vi "HFRR ADV v044.vi"() -> ()   [LabVIEW 2025] (continued)
                n2757 = Multiply(x=w3274, y=w3260) -> (x*y=w3266:dbl)
                n2758 = Subtract(x=w3267, y=w3277) -> (x-y=w3269:dbl)
                n2759 = local read "Save"() -> (w3270:bool)
                n2760 = Add(x=w3269, y=w3266) -> (x+y=w3253:dbl)
                "Elapsed time 3" <- w3253
                n2761 = And(x=w3255, y=w3270) -> (x .and. y?=w3268:bool)
                n2762 = Divide(x=w3253, y=60.0) -> (x/y=w3264:dbl)
                n2763 = local read "Test \nStatus"() -> (w3254:bool)
                n2764 = local read "clk"() -> (w3261:dbl)
                n2765 = Equal?(x=w3261, y=10.0) -> (x = y?=w3263:bool)
                n2766 = case shown="True" w3268 {
                  tunnel: w3267 -> [_ w3394]
                  tunnel: [FALSE ("Boolean 2") TRUE ("Boolean 2")] -> _
                  frame False {
                  }
                  frame True {
                    w3348 = ";" ("Substring")
                    # "Pid out/\nFreq response value"
                    n2767 = local write "act save time"(w3394) -> ()
                    n2768 = local read "FILE"() -> (w3342:string)
                    n2769 = call "file check.vi"("file name in"=w3342) -> ("error out"=w3345:errorcluster, "file name out"=w3340:string)  [unwired: 9 in]
                    n2770 = local read "LVDT STROKE"() -> (w3337:dbl)
                    n2771 = local read "Add up Stroke"() -> (w3335:dbl)
                    n2772 = call "FILE PATH CREATION.vi"("error in"=w3345, "FILE NAME :"=w3340) -> ("FILE OUT"=w3343:path)  [unwired: 8 in, 1 out]
                    n2773 = local read "STROKE Initialize"() -> (w3330:bool)
                    n2774 = Concatenate Strings(w3340, ".dgf" ("Substring")) -> (w3344:string)
                    n2775 = Subtract(x=w3337, y=w3335) -> (x-y=w3336:dbl)
                    n2776 = Absolute Value(x=w3336) -> (abs(x)=w3333:dbl)
                    n2777 = local read "FF 2"() -> (→"Frictional Force ( N )" →"Frictional Force ( N )":dbl)
                    n2778 = Build Path(base path=w3343, name or relative path=w3344) -> (appended path=w3339:path)
                    n2779 = flat-sequence {
                      tunnel: w3333 -> [w3399]
                      tunnel: [w3398] -> w3331
                      tunnel: w3330 -> [w3396]
                      tunnel: [w3401] -> w3332
                      tunnel: w3331 -> [w3401]
                      frame #0 {
                        n2780 = call <vilib>:"Mean PtByPt.vi"("x"=w3399, "sample length"="STROKE FILTER", "initialize"=w3396) -> ("mean"=w3398:dbl)  [unwired: 1 in, 1 out]
                      }
                      frame #1 {
                        "STROKE Initialize" <- FALSE ("STROKE Initialize")
                      }
                    }
                    n2781 = local read "COF 2"() -> (w3353:dbl)
                    "Coefficient of Friction" <- w3353
                    "COF 4" <- w3353
                    "Coefficient of Friction" <- w3353
                    n2782 = local read "TEMP"() -> (w3356:dbl)
                    "Temperature ( Deg C )" <- w3356
                    n2783 = local read "Humidity ( %RH )"() -> (w3355:dbl)
                    n2784 = local read "Frequency ( Hz )"() -> (w3362:dbl)
                    n2785 = local read "LVDT STROKE DISPLAY"() -> (w3334:dbl)
                    n2786 = local read "Elapsed time"() -> (w3387:dbl)
                    n2787 = local read "AIR TEMP"() -> (w3360:dbl)
                    n2788 = local read "PID-out"() -> (w3365:dbl)
                    n2789 = local write "Temperature ( Deg C )"(w3356) -> ()
                    n2790 = Number To Fractional String(number=w3334, width (-)=i16 9 ("precision (6)"), precision (6)=i16 6) -> (F-format string=w3380:string)  [unwired: 1 in]
                    n2791 = Number To Fractional String(number=w3360, width (-)=i16 9 ("precision (6)"), precision (6)=i16 3) -> (F-format string=w3379:string)  [unwired: 1 in]
                    n2792 = Number To Fractional String(number=w3356, width (-)=i16 9 ("precision (6)"), precision (6)=i16 3) -> (F-format string=w3376:string)  [unwired: 1 in]
                    n2793 = Number To Fractional String(number=w3355, width (-)=i16 9 ("precision (6)"), precision (6)=i16 3) -> (F-format string=w3373:string)  [unwired: 1 in]
                    n2794 = Number To Fractional String(number=0.0, width (-)=i16 9 ("precision (6)"), precision (6)=i16 3) -> (F-format string=w3370:string)  [unwired: 1 in]
                    n2795 = Number To Fractional String(number=w3365, width (-)=i16 9 ("precision (6)"), precision (6)=i16 3) -> (F-format string=w3366:string)  [unwired: 1 in]
                    n2796 = Number To Fractional String(number=w3362, width (-)=i16 9 ("precision (6)"), precision (6)=i16 3) -> (F-format string=w3361:string)  [unwired: 1 in]
                    n2797 = Number To Fractional String(number=w3353, width (-)=i16 9 ("precision (6)"), precision (6)=i16 6) -> (F-format string=w3388:string)  [unwired: 1 in]
                    n2798 = Number To Fractional String(number=w3387, width (-)=i16 14 ("precision (6)"), precision (6)=i16 3) -> (F-format string=w3389:string)  [unwired: 1 in]
                    n2799 = Bundle("y"=1.02, "LVDT STROKE DISPLAY"=w3334, "y"=0.98) -> (w3354:T30)  [unwired: 1 in]
                    n2800 = Number To Fractional String(number="Ambient Humidity :", width (-)=i16 9 ("precision (6)"), precision (6)=i16 6) -> (F-format string=w3346:string)  [unwired: 1 in]
                    n2801 = local read "RUN"() -> (w3352:bool)
                    n2802 = case shown="True" w3352 {
                      tunnel: w3354 -> [_ w3405]
                      tunnel: w3334 -> [_ w3404]
                      tunnel: w3334 -> [_ w3402]
                      tunnel: w3334 -> [_ w3403]
                      frame False {
                      }
                      frame True {
                        "Stroke ( mm )" <- w3405
                        "Stroke ( mm )" <- w3405
                        "Stroke 4" <- w3404
                        "Stroke 3" <- w3402
                        "Stroke 2" <- w3403
                        "measured_stroke" <- w3402
                      }
                    }
                    n2803 = Concatenate Strings(w3389, w3348, w3388, w3348, w3380, w3348, w3379, w3348, w3376, w3348, w3373, w3348, w3370, w3348, w3366, w3348, w3361, w3348, w3346, "\r") -> (w3386:string)
                    n2804 = call <vilib>:"Write Characters To File.vi"("append to file? (new file:F)"=TRUE, "character string"=w3386, "file path (dialog if empty)"=w3339) -> ()  [unwired: 2 in, 1 out]
                    "refresh flag" <- TRUE ("refresh flag")
                    "LVDT STROKE Actual" <- w3332
                  }
                }
                n2805 = case shown="True" w3254 {
                  tunnel: w3264 -> [_ w3290]
                  tunnel: w3269 -> [_ w3300]
                  tunnel: [0.0 w3296] -> _
                  tunnel: w3263 -> [_ w3295]
                  tunnel: [0.0 w3294] -> _
                  tunnel: w3253 -> [_ w3294]
                  tunnel: w3267 -> [w3283 _]
                  frame False {
                    n2806 = local write "acq timer"(w3283) -> ()
                    n2807 = local write "Test Duration Status"(0.0 ("Test Duration Status")) -> ()
                  }
                  frame True {
                    n2808 = local read "Set Hz"() -> (w3297:dbl)
                    n2809 = local write "Elapsed time"(w3290) -> ()
                    n2810 = local read "test time"() -> (w3289:dbl)
                    n2811 = Multiply(x=w3300, y=w3297) -> (x*y=w3299:dbl)
                    n2812 = case shown="False" w3295 {
                      tunnel: w3299 -> [w3301 _]
                      tunnel: [w3301 1.0] -> w3296
                      frame False {
                        n2813 = local write "Cycles elapsed"(w3301) -> ()
                      }
                      frame True {
                      }
                    }
                    n2814 = Greater?(x=w3290, y=w3289) -> (0:w3298:bool)
                    n2815 = Subtract(x=w3289, y=w3290) -> (x-y=w3288:dbl)
                    n2816 = Multiply(x=w3288, y=60.0) -> (x*y=w3287:dbl)
                    n2817 = local write "Time Remaining"(w3287) -> ()
                    n2818 = local write "Remaining Time"(w3287) -> ()
                    n2819 = case shown="True" w3298 {
                      frame False {
                      }
                      frame True {
                        n2820 = stacked-sequence {
                          frame #0 {
                            w3306 = T19."Enabled" ("Disabled")
                            w3305 = FALSE ("TEST FILE NAM,E SAVED")
                            w3307 = "" ("FILE")
                            w3308 = TRUE ("Visible")
                            n2821 = local write "Humidity"(FALSE ("Humidity")) -> ()
                            n2822 = local write "RUN"(FALSE ("OK Button 2")) -> ()
                            n2823 = local write "Heater Button"(FALSE ("Heater Button")) -> ()
                            n2824 = local write "Auto Start Test"(FALSE ("Auto Start Test")) -> ()
                            n2825 = local write "TestCompFlg"(TRUE ("StpFlg")) -> ()
                            n2826 = local read "Humidity ( %RH )"() -> (→"Rh After":dbl)
                            n2827 = property on="STOP 2" class="Bool (strict)"("Disabled"=u8 0) -> ()  [unwired: 2 in, 2 out]
                            n2828 = local read "EVENT LOG"() -> (w3313:string)
                            n2829 = call "Event Log.vi"("Content"="Test Completed", "EVENT LOG"=w3313) -> ("EVENT LOG"=w3312:string)  [unwired: 8 in, 1 out]
                            n2830 = property on="RUN" class="Bool (strict)"("Visible"=w3308) -> ()  [unwired: 2 in, 2 out]
                            n2831 = property on="Auto Start Test" class="Bool (strict)"("Visible"=w3308) -> ()  [unwired: 2 in, 2 out]
                            n2832 = local write "Batch Ref Num :"(w3307) -> ()
                            n2833 = local write "FILE"(w3307) -> ()
                            n2834 = local write "EVENT LOG"(w3312) -> ()
                            n2835 = local write "TEST FILE NAM,E SAVED"(w3305) -> ()
                            n2836 = local write "Fuel Discription :"(w3307) -> ()
                            n2837 = local write "START TEMP"(w3305) -> ()
                            n2838 = local write "Remarks :"(w3307) -> ()
                            n2839 = local write "Main Dashboard Buttons"(T1."Imaging" ("Main Dashboard Buttons")) -> ()
                            n2840 = local write "Main Tab"(T4."Adv Scar" ("Main Tab")) -> ()
                            n2841 = property on="FRICVALZ 2" class="Bool (strict)"("DisabledEnum"=w3306) -> ()  [unwired: 2 in, 2 out]
                            n2842 = property on="FRICVALZ 3" class="Bool (strict)"("DisabledEnum"=w3306) -> ()  [unwired: 2 in, 2 out]
                            n2843 = property on="FRICVALZ 4" class="Bool (strict)"("DisabledEnum"=w3306) -> ()  [unwired: 2 in, 2 out]
                          }
                          frame #1 {
                            n2844 = Wait (ms)(milliseconds to wait=u32 2000) -> ()  [unwired: 1 out]
                          }
                          frame #2 {
                            n2845 = local write "Due Write"("VC;0") -> ()
                          }
                          frame #3 {
                            n2846 = Wait (ms)(milliseconds to wait=u32 2000) -> ()  [unwired: 1 out]
                          }
                          frame #4 {
                            n2847 = local write "Due Write"("VC;0") -> ()
                          }
                          frame #5 {
                            n2848 = Wait (ms)(milliseconds to wait=u32 2000) -> ()  [unwired: 1 out]
                          }
                          frame #6 {
                            n2849 = local write "Due Write"("ST;0") -> ()
                          }
                          frame #7 {
                            n2850 = local write "measured_stroke"(0.0 ("measured_stroke")) -> ()
                            n2851 = Wait (ms)(milliseconds to wait=u32 1500) -> ()  [unwired: 1 out]
                          }
                          frame #8 {
                            n2852 = local write "Due Write"("HE;0") -> ()
                            n2853 = local write "Humidity 2"(TRUE ("Humidity")) -> ()
                          }
                        }
                      }
                    }
                    n2854 = Divide(x=w3290, y=w3289) -> (x/y=w3293:dbl)
                    n2855 = Multiply(x=w3293, y=100.0) -> (x*y=w3291:dbl)
                    n2856 = local write "Test Duration Status"(w3291) -> ()
                  }
                }
              }
              frame #2 {
                n2857 = case shown="True" "Heater Button" {
                  tunnel: [0.0 ("output") w3428] -> w3406
                  frame False {
                    w3409 = TRUE ("tmpchk")
                    n2858 = local read "TEMP"() -> (w3410:dbl)
                    n2859 = local write "Temp ini"(w3410) -> ()
                    n2860 = local write "Reset 4"(w3409) -> ()
                    n2861 = local write "tmpchk"(w3409) -> ()
                    n2862 = local write "reinit"(TRUE ("reinit")) -> ()
                    n2863 = local write "manual temp log"(TRUE ("manual temp log")) -> ()
                  }
                  frame True {
                    # "Logic to turn off\nthe heater when \ntemp is not rising.\nTime - 60 sec\nDelta t- 5°c"
                    n2864 = local read "Temp ini"() -> (w3417:dbl)
                    n2865 = local read "Auto Start Test"() -> (w3413:bool)
                    n2866 = Less?(x=w3417, y=53.0) -> (x < y?=w3415:bool)
                    n2867 = case shown="False" w3413 {
                      frame False {
                        n2868 = local read "Set Temp"() -> (w3437:dbl)
                        n2869 = local read "TEMP"() -> (w3436:dbl)
                        n2870 = Subtract(x=w3437, y=w3436) -> (x-y=w3435:dbl)
                        n2871 = Absolute Value(x=w3435) -> (abs(x)=w3434:dbl)
                        n2872 = Less?(x=w3434, y=0.5) -> (x < y?=w3432:bool)
                        n2873 = case shown="True" w3432 {
                          tunnel: "manual temp log" -> [_ w3438]
                          frame False {
                          }
                          frame True {
                            n2874 = case shown="True" w3438 {
                              selector: w3438 -> [_ w3439]
                              frame False {
                              }
                              frame True {
                                # "#Event log"
                                n2875 = Not(x=w3439) -> (.not. x?=w3440:bool)
                                n2876 = local write "manual temp log"(w3440) -> ()
                                n2877 = local read "EVENT LOG"() -> (w3443:string)
                                n2878 = call "Event Log.vi"("Content"="Target Temperature reached", "EVENT LOG"=w3443) -> ("EVENT LOG"=w3442:string)  [unwired: 8 in, 1 out]
                                n2879 = local write "EVENT LOG"(w3442) -> ()
                              }
                            }
                          }
                        }
                      }
                      frame True {
                        n2880 = local write "manual temp log"(TRUE ("manual temp log")) -> ()
                      }
                    }
                    n2881 = And(x="tmpchk", y=w3415) -> (x .and. y?=w3418:bool)
                    n2882 = case shown="True" w3418 {
                      frame False {
                      }
                      frame True {
                        n2883 = call "Elapsed Time8"("Time Target (s)"=300.0, "Reset"="Reset 4") -> ("Time has Elapsed"=w3445:bool)  [unwired: 10 in, 7 out]
                        n2884 = flat-sequence {
                          tunnel: w3445 -> [_]
                          frame #0 {
                            n2885 = local write "Reset 4"(FALSE ("Reset 4")) -> ()
                          }
                        }
                        n2886 = case shown="True" w3445 {
                          frame False {
                          }
                          frame True {
                            n2887 = local read "Temp ini"() -> (w3452:dbl)
                            n2888 = Add(x=w3452, y=5.0) -> (x+y=w3450:dbl)
                            n2889 = local read "TEMP"() -> (w3453:dbl)
                            n2890 = Greater?(x=w3453, y=w3450) -> (0:w3451:bool)
                            n2891 = case shown="False" w3451 {
                              frame False {
                                n2892 = local write "Heater Button"(FALSE ("Heater Button")) -> ()
                              }
                              frame True {
                                n2893 = local write "tmpchk"(FALSE ("tmpchk")) -> ()
                              }
                            }
                          }
                        }
                      }
                    }
                    n2894 = local read "Set Temp"() -> (w3426:dbl)
                    n2895 = local read "TEMP"() -> (w3420:dbl)
                    n2896 = call-poly <vilib>:"PID.vi"("reinitialize? (F)"="reinit", "dt (s)"=-1.0, "process variable"=w3420, "setpoint"=w3426) -> ("output"=w3423:dbl)  [unwired: 6 in, 1 out]
                    n2897 = Subtract(x=w3426, y=w3420) -> (x-y=w3427:dbl)
                    n2898 = Add(x=w3426, y=0.5) -> (x+y=w3424:dbl)
                    n2899 = Greater Or Equal?(x=w3420, y=w3424) -> ()  [unwired: 1 out]
                    n2900 = Select(t=0.0, s=FALSE, f=w3423) -> (s? t:f=w3422:dbl)
                    "PID output" <- w3422
                    n2901 = flat-sequence {
                      tunnel: w3422 -> [w3456]
                      tunnel: [w3456] -> w3428
                      frame #0 {
                        n2902 = local write "reinit"(FALSE ("reinit")) -> ()
                      }
                    }
                    n2903 = Bundle(w3427, "output"=w3422, "TEMP"=w3420) -> ()  [unwired: 1 in, 1 out]
                  }
                }
                "PID-out" <- w3406
              }
              frame #3 {
                n2904 = local read "TEMP"() -> (w3458:dbl)
                n2905 = Greater Or Equal?(x=w3458, y="Set Temp 2") -> (x >= y?=w3463:bool)
                n2906 = case shown="True" w3463 {
                  tunnel: [FALSE TRUE] -> w3461
                  frame False {
                  }
                  frame True {
                  }
                }
                "Status 13" <- w3461
                n2907 = And(x=w3461, y="trip1 8") -> (x .and. y?=w3460:bool)
                n2908 = case shown="True" w3460 {
                  frame False {
                    n2909 = local write "Heater Trip Temp"(TRUE ("Heater Trip Temp")) -> ()
                  }
                  frame True {
                    w3466 = FALSE ("OK Button 2")
                    n2910 = case shown="True" "Heater Trip Temp" {
                      selector: "Heater Trip Temp" -> [_ w3468]
                      frame False {
                      }
                      frame True {
                        n2911 = Not(x=w3468) -> (.not. x?=w3467:bool)
                        n2912 = local read "EVENT LOG"() -> (w3471:string)
                        n2913 = local write "Heater Trip Temp"(w3467) -> ()
                        n2914 = call "Event Log.vi"("Content"="Heater Trip", "EVENT LOG"=w3471) -> ("EVENT LOG"=w3470:string)  [unwired: 8 in, 1 out]
                        n2915 = local write "EVENT LOG"(w3470) -> ()
                      }
                    }
                    n2916 = local write "RUN"(w3466) -> ()
                    n2917 = property on="Auto Start Test" class="Bool (strict)"("Value"=w3466) -> ()  [unwired: 2 in, 2 out]
                    n2918 = local write "Heater Button"(w3466) -> ()
                  }
                }
              }
            }
            n2919 = case shown="False" w3177 {
              frame False {
                n2920 = disable-structure shown="Disabled" {
                  frame Disabled {
                    n2921 = stacked-sequence {
                      frame #0 {
                        n2922 = local write "RUN"(FALSE ("OK Button 2")) -> ()
                      }
                      frame #1 {
                      }
                    }
                  }
                  frame Enabled {
                  }
                }
              }
              frame True {
              }
            }
          }
        }
        n2923 = local read "Reset Graph"() -> (w3074:bool)
        n2924 = case shown="True" w3074 {
          selector: w3074 -> [_ w3091]
          frame False {
          }
          frame True {
            w3105 = 0.0 ("X Scale.Range:Maximum")
            n2925 = Not(x=w3091) -> (.not. x?=w3090:bool)
            n2926 = local write "Reset Graph"(w3090) -> ()
            n2927 = property on="Electrical Contact Resistance ( % )" class="WFChart (strict)"("XScale.Maximum"=600.0 ("X Scale.Range:Maximum"), "XScale.Minimum"=0.0 ("X Scale.Range:Minimum"), "YScale.Maximum"=100.0 ("Y Scale.Range:Maximum"), "YScale.Minimum"=0.0 ("Y Scale.Range:Minimum")) -> ()  [unwired: 2 in, 2 out]
            n2928 = property on="Frictional Force ( N )" class="WFChart (strict)"("XScale.Maximum"=600.0 ("X Scale.Range:Maximum"), "XScale.Minimum"=0.0 ("X Scale.Range:Minimum"), "YScale.Maximum"=100.0 ("Y Scale.Range:Maximum"), "YScale.Minimum"=0.0 ("Y Scale.Range:Minimum")) -> ()  [unwired: 2 in, 2 out]
            n2929 = property on="Temperature ( Deg C )" class="WFChart (strict)"("XScale.Maximum"=600.0 ("X Scale.Range:Maximum"), "XScale.Minimum"=0.0 ("X Scale.Range:Minimum"), "YScale.Maximum"=100.0 ("Y Scale.Range:Maximum"), "YScale.Minimum"=0.0 ("Y Scale.Range:Minimum")) -> ()  [unwired: 2 in, 2 out]
            n2930 = property on="Stroke ( mm )" class="WFChart (strict)"("XScale.Maximum"=600.0 ("X Scale.Range:Maximum"), "XScale.Minimum"=0.0 ("X Scale.Range:Minimum"), "YScale.Maximum"=100.0 ("Y Scale.Range:Maximum"), "YScale.Minimum"=0.0 ("Y Scale.Range:Minimum")) -> ()  [unwired: 2 in, 2 out]
            n2931 = property on="Coefficient of Friction" class="WFChart (strict)"("XScale.Maximum"=600.0 ("X Scale.Range:Maximum"), "XScale.Minimum"=0.0 ("X Scale.Range:Minimum"), "YScale.Maximum"=100.0 ("Y Scale.Range:Maximum"), "YScale.Minimum"=0.0 ("Y Scale.Range:Minimum")) -> ()  [unwired: 2 in, 2 out]
            n2932 = property on="Electrical Contact Resistance ( % )" class="WFChart (strict)"("XScale.Minimum"=0.0 ("X Scale.Range:Minimum"), "XScale.Maximum"=600.0 ("X Scale.Range:Maximum"), "YScale.Minimum"=0.0 ("Y Scale.Range:Minimum"), "YScale.Maximum"=100.0 ("Y Scale.Range:Maximum")) -> ()  [unwired: 2 in, 2 out]
            n2933 = property on="Temperature ( Deg C )" class="WFChart (strict)"("XScale.Minimum"=0.0 ("X Scale.Range:Minimum"), "XScale.Maximum"=600.0 ("X Scale.Range:Maximum"), "YScale.Minimum"=0.0 ("Y Scale.Range:Minimum"), "YScale.Maximum"=100.0 ("Y Scale.Range:Maximum")) -> ()  [unwired: 2 in, 2 out]
            n2934 = property on="Coefficient of Friction" class="WFChart (strict)"("XScale.Minimum"=0.0 ("X Scale.Range:Minimum"), "XScale.Maximum"=600.0 ("X Scale.Range:Maximum"), "YScale.Maximum"=1.0 ("X Scale.Range:Minimum"), "YScale.Minimum"=0.0 ("X Scale.Range:Minimum")) -> ()  [unwired: 2 in, 2 out]
            n2935 = property on="Frictional Force ( N )" class="WFChart (strict)"("XScale.Maximum"=600.0 ("X Scale.Range:Maximum"), "XScale.Minimum"=w3105, "YScale.Maximum"=10.0 ("Y Scale.Range:Maximum"), "YScale.Minimum"=w3105) -> ()  [unwired: 2 in, 2 out]
            n2936 = property on="Stroke ( mm )" class="WFChart (strict)"("XScale.Maximum"=600.0 ("X Scale.Range:Maximum"), "XScale.Minimum"=0.0 ("X Scale.Range:Minimum"), "YScale.Maximum"=100.0 ("Y Scale.Range:Maximum"), "YScale.Minimum"=0.0 ("Y Scale.Range:Minimum")) -> ()  [unwired: 2 in, 2 out]
          }
        }
      }
      frame "Compare Files" {
        # "Elapsed time\ncof\nstroke\nAir temp\nTemp\nHumidity"
        n2937 = case shown="True" "RSTV1 2" {
          frame False {
          }
          frame True {
            n2938 = property on="Humidity ( %RH )" class="XYGraph (strict)"("Y Scale.Display Format:Precision"=u8 0 ("Y Scale.Format & Precision:Precision")) -> ()  [unwired: 2 in, 2 out]
            n2939 = property on="Humidity ( %RH )" class="XYGraph (strict)"("X Scale.Range:Minimum"=0.0, "X Scale.Range:Maximum"=75.0, "Y Scale.Range:Minimum"=48.0, "Y Scale.Range:Maximum"=58.0) -> ()  [unwired: 2 in, 2 out]
          }
        }
        n2940 = case shown="True" "RST CP 2" {
          frame False {
          }
          frame True {
            n2941 = property on="XY Graph 13" class="XYGraph (strict)"("Y Scale.Display Format:Precision"=u8 0 ("Y Scale.Format & Precision:Precision")) -> ()  [unwired: 2 in, 2 out]
            n2942 = property on="XY Graph 13" class="XYGraph (strict)"("X Scale.Range:Minimum"=0.0, "X Scale.Range:Maximum"=75.0, "Y Scale.Range:Minimum"=0.0, "Y Scale.Range:Maximum"=100.0) -> ()  [unwired: 2 in, 2 out]
          }
        }
        n2943 = case shown="True" "RST CP" {
          frame False {
          }
          frame True {
            n2944 = property on="Sample Temperature ( °C )" class="XYGraph (strict)"("Y Scale.Display Format:Precision"=u8 2 ("Y Scale.Format & Precision:Precision")) -> ()  [unwired: 2 in, 2 out]
            n2945 = property on="Sample Temperature ( °C )" class="XYGraph (strict)"("X Scale.Range:Minimum"=0.0, "X Scale.Range:Maximum"=75.0, "Y Scale.Range:Minimum"=58.0, "Y Scale.Range:Maximum"=62.0) -> ()  [unwired: 2 in, 2 out]
          }
        }
        n2946 = case shown="True" "RSTV1 3" {
          frame False {
          }
          frame True {
            n2947 = property on="Air Temperature  ( °C )" class="XYGraph (strict)"("Y Scale.Display Format:Precision"=u8 2 ("Y Scale.Format & Precision:Precision")) -> ()  [unwired: 2 in, 2 out]
            n2948 = property on="Air Temperature  ( °C )" class="XYGraph (strict)"("X Scale.Range:Minimum"=0.0 ("Y Scale.Range:Minimum"), "X Scale.Range:Maximum"=75.0 ("Y Scale.Range:Maximum"), "Y Scale.Range:Minimum"=20.0 ("X Scale.Range:Minimum"), "Y Scale.Range:Maximum"=26.0 ("X Scale.Range:Maximum")) -> ()  [unwired: 2 in, 2 out]
          }
        }
        n2949 = case shown="True" "RSTV1 4" {
          frame False {
          }
          frame True {
            n2950 = property on="Stroke ( mm )" class="XYGraph (strict)"("Y Scale.Display Format:Precision"=u8 2 ("Y Scale.Format & Precision:Precision")) -> ()  [unwired: 2 in, 2 out]
            n2951 = property on="Stroke ( mm )" class="XYGraph (strict)"("X Scale.Range:Minimum"=0.0 ("Y Scale.Range:Maximum"), "X Scale.Range:Maximum"=75.0 ("X Scale.Range:Minimum"), "Y Scale.Range:Minimum"=0.98, "Y Scale.Range:Maximum"=1.02) -> ()  [unwired: 2 in, 2 out]
          }
        }
        n2952 = case shown="True" "rstv2" {
          frame False {
          }
          frame True {
            n2953 = property on="Coefficient Of Friction" class="XYGraph (strict)"("Y Scale.Display Format:Precision"=u8 3 ("Y Scale.Format & Precision:Precision")) -> ()  [unwired: 2 in, 2 out]
            n2954 = property on="Coefficient Of Friction" class="XYGraph (strict)"("X Scale.Range:Minimum"=0.0 ("Y Scale.Range:Maximum"), "X Scale.Range:Maximum"=75.0, "Y Scale.Range:Minimum"=0.0, "Y Scale.Range:Maximum"=1.0 ("X Scale.Range:Minimum")) -> ()  [unwired: 2 in, 2 out]
          }
        }
        n2955 = case shown="True" "RST CP 3" {
          frame False {
          }
          frame True {
            n2956 = property on="Air Temp ( °C ) vs Humidity ( % RH )" class="XYGraph (strict)"("X Scale.Range:Minimum"=18.0, "X Scale.Range:Maximum"=28.0 ("X Scale.Range:Minimum"), "Y Scale.Range:Minimum"=30.0 ("X Scale.Range:Minimum"), "Y Scale.Range:Maximum"=70.0 ("X Scale.Range:Minimum")) -> ()  [unwired: 2 in, 2 out]
          }
        }
        n2957 = case shown="True" "OPEN 1" {
          frame False {
          }
          frame True {
            (unwired) 0  # existing file
            w3747 = "Choose a datalog file to open"  # prompt
            n2958 = local write "OPEN 1"(FALSE ("OPEN 1")) -> ()
            n2959 = String To Path(string="C:\\LAB-IQ\\Data\\") -> (path=w3732:path)
            n2960 = File Dialog(6:"*.dgf" ("pattern"), 7:w3747, 11:w3732) -> (0:w3730:errorcluster, 3:w3738:path)  [unwired: 4 in, 2 out]
            n2961 = Unbundle(w3730) -> ()  [unwired: 3 out]
            n2962 = Strip Path(path=w3738) -> (name=w3737:string)  [unwired: 1 out]
            n2963 = Path To String(path=w3738) -> (string=w3733:string)
            "string1" <- w3733
            n2964 = Match Pattern(string=w3737, regular expression=".dgf") -> (before substring=→"String Control":string)  [unwired: 1 in, 3 out]
            n2965 = Match Pattern(string=w3733, regular expression=".dgf" ("substring (\"\")")) -> (before substring=w3743:string)  [unwired: 1 in, 3 out]
            n2966 = Concatenate Strings(w3743, ".duf" ("Substring")) -> (w3739:string)
            n2967 = String To Path(string=w3739) -> (path=w3744:path)
            n2968 = call <vilib>:"Read Characters From File.vi"("file path (dialog if empty)"=w3744, "start of read offset (chars.:0)"=60 ("start of read offset (chars.: 0)")) -> ("character string"=→"String Control 2":string)  [unwired: 4 in, 3 out]
          }
        }
        n2969 = case shown="True" "OPEN 2" {
          frame False {
          }
          frame True {
            (unwired) 0  # existing file
            w3765 = "Choose a datalog file to open"  # prompt
            n2970 = local write "OPEN 2"(FALSE ("OPEN 1")) -> ()
            n2971 = String To Path(string="C:\\LAB-IQ\\Data\\") -> (path=w3750:path)
            n2972 = File Dialog(6:"*.dgf" ("pattern"), 7:w3765, 11:w3750) -> (0:w3748:errorcluster, 3:w3756:path)  [unwired: 4 in, 2 out]
            n2973 = Unbundle(w3748) -> ()  [unwired: 3 out]
            n2974 = Strip Path(path=w3756) -> (name=w3754:string)  [unwired: 1 out]
            n2975 = Path To String(path=w3756) -> (string=w3751:string)
            "string1 2" <- w3751
            n2976 = Match Pattern(string=w3754, regular expression=".dgf") -> (before substring=→"String Control 3":string)  [unwired: 1 in, 3 out]
            n2977 = Match Pattern(string=w3751, regular expression=".dgf" ("substring (\"\")")) -> (before substring=w3762:string)  [unwired: 1 in, 3 out]
            n2978 = Concatenate Strings(w3762, ".duf" ("Substring")) -> (w3759:string)
            n2979 = String To Path(string=w3759) -> (path=w3757:path)
            n2980 = call <vilib>:"Read Characters From File.vi"("file path (dialog if empty)"=w3757, "start of read offset (chars.:0)"=60 ("start of read offset (chars.: 0)")) -> ("character string"=→"String Control 4":string)  [unwired: 4 in, 3 out]
          }
        }
        n2981 = case shown="True" "OPEN 3" {
          frame False {
          }
          frame True {
            (unwired) 0  # existing file
            w3783 = "Choose a datalog file to open"  # prompt
            n2982 = local write "OPEN 3"(FALSE ("OPEN 1")) -> ()
            n2983 = String To Path(string="C:\\LAB-IQ\\Data\\") -> (path=w3768:path)
            n2984 = File Dialog(6:"*.dgf" ("pattern"), 7:w3783, 11:w3768) -> (0:w3766:errorcluster, 3:w3774:path)  [unwired: 4 in, 2 out]
            n2985 = Unbundle(w3766) -> ()  [unwired: 3 out]
            n2986 = Strip Path(path=w3774) -> (name=w3772:string)  [unwired: 1 out]
            n2987 = Path To String(path=w3774) -> (string=w3769:string)
            "string1 3" <- w3769
            n2988 = Match Pattern(string=w3772, regular expression=".dgf") -> (before substring=→"String Control 5":string)  [unwired: 1 in, 3 out]
            n2989 = Match Pattern(string=w3769, regular expression=".dgf" ("substring (\"\")")) -> (before substring=w3779:string)  [unwired: 1 in, 3 out]
            n2990 = Concatenate Strings(w3779, ".duf" ("Substring")) -> (w3776:string)
            n2991 = String To Path(string=w3776) -> (path=w3780:path)
            n2992 = call <vilib>:"Read Characters From File.vi"("file path (dialog if empty)"=w3780, "start of read offset (chars.:0)"=60 ("start of read offset (chars.: 0)")) -> ("character string"=→"String Control 6":string)  [unwired: 4 in, 3 out]
          }
        }
        n2993 = case shown="True" "OPEN 4" {
          frame False {
          }
          frame True {
            (unwired) 0  # existing file
            w3801 = "Choose a datalog file to open"  # prompt
            n2994 = local write "OPEN 4"(FALSE ("OPEN 1")) -> ()
            n2995 = String To Path(string="C:\\LAB-IQ\\Data\\") -> (path=w3786:path)
            n2996 = File Dialog(6:"*.dgf" ("pattern"), 7:w3801, 11:w3786) -> (0:w3784:errorcluster, 3:w3792:path)  [unwired: 4 in, 2 out]
            n2997 = Unbundle(w3784) -> ()  [unwired: 3 out]
            n2998 = Strip Path(path=w3792) -> (name=w3790:string)  [unwired: 1 out]
            n2999 = Path To String(path=w3792) -> (string=w3787:string)
            "string1 4" <- w3787
            n3000 = Match Pattern(string=w3790, regular expression=".dgf") -> (before substring=→"String Control 7":string)  [unwired: 1 in, 3 out]
            n3001 = Match Pattern(string=w3787, regular expression=".dgf" ("substring (\"\")")) -> (before substring=w3797:string)  [unwired: 1 in, 3 out]
            n3002 = Concatenate Strings(w3797, ".duf" ("Substring")) -> (w3794:string)
            n3003 = String To Path(string=w3794) -> (path=w3798:path)
            n3004 = call <vilib>:"Read Characters From File.vi"("file path (dialog if empty)"=w3798, "start of read offset (chars.:0)"=60 ("start of read offset (chars.: 0)")) -> ("character string"=→"String Control 8":string)  [unwired: 4 in, 3 out]
          }
        }
      }
      frame "About" {
        # "Elapsed time\ncof\nstroke\nmean pos\nTemp\nHumidity"
        n3005 = disable-structure shown="Disabled" {
          frame Disabled {
            n3006 = case shown="True" "Export" {
              frame False {
              }
              frame True {
                w3823 = "                                      " ("string")
                w3825 = "\r"
                (unwired) i16 6 ("width (-)")
                w3902 = "\r"
                w3834 = "\r"
                n3007 = local write "Export"(FALSE ("Export")) -> ()
                n3008 = local read "String 29"() -> (w3871:string)
                n3009 = local read "String 34"() -> (w3859:string)
                n3010 = local read "String 35"() -> (w3854:string)
                n3011 = local read "String 37"() -> (w3850:string)
                n3012 = local read "String 36"() -> (w3847:string)
                n3013 = local read "String 38"() -> (w3844:string)
                n3014 = local read "String 39"() -> (w3841:string)
                n3015 = Match Pattern(string=w3871, regular expression=".dwm") -> (before substring=w3867:string)  [unwired: 1 in, 3 out]
                "before substring" <- w3867
                n3016 = local read "S 38"() -> (w3862:string)
                n3017 = local read "S 39"() -> (w3855:string)
                n3018 = local read "Temperature before test 2"() -> (w3891:dbl)
                n3019 = local read "Temperature after test 2"() -> (w3896:dbl)
                n3020 = local read "Humidity before test 2"() -> (w3877:dbl)
                n3021 = local read "Humidity after test 2"() -> (w3892:dbl)
                n3022 = local read "MWSD 2"() -> (w3888:dbl)
                n3023 = local read "WS1.4 2"() -> (w3904:dbl)
                n3024 = local read "HCF 2"() -> (w3900:dbl)
                n3025 = local read "AVP 2"() -> (w3889:dbl)
                n3026 = Concatenate Strings("1," ("string"), w3862) -> (w3861:string)
                n3027 = Concatenate Strings("2," ("string"), w3859) -> (w3858:string)
                n3028 = Concatenate Strings("3," ("string"), w3855) -> (w3857:string)
                n3029 = Concatenate Strings("4," ("string"), w3854) -> (w3853:string)
                n3030 = Concatenate Strings("5," ("string"), w3850) -> (w3851:string)
                n3031 = Concatenate Strings("6," ("string"), w3847) -> (w3848:string)
                n3032 = Concatenate Strings("7," ("string"), w3844) -> (w3845:string)
                n3033 = Concatenate Strings("8," ("string"), w3841) -> (w3842:string)
                n3034 = local read "Sample ID"() -> (w3909:string)
                n3035 = case shown="\"xlx\"" "Select File Type" {
                  tunnel: w3867 -> [w3912 w3914 w3916]
                  tunnel: [w3910 w3915 w3917] -> w3866
                  frame "xlx" {
                    n3036 = Concatenate Strings(w3912, ".xls" ("string")) -> (w3910:string)
                  }
                  frame "csv" {
                    n3037 = Concatenate Strings(w3914, ".csv" ("string")) -> (w3915:string)
                  }
                  frame "txt" {
                    n3038 = Concatenate Strings(w3916, ".txt" ("string")) -> (w3917:string)
                  }
                }
                n3039 = local read "Test Date"() -> (w3908:string)
                n3040 = local read "String 45"() -> (w3822:string)
                n3041 = local read "String 31"() -> (w3907:string)
                n3042 = local read "String 32"() -> (w3906:string)
                n3043 = local read "TITTLE"() -> (w3830:string)
                n3044 = Number To Fractional String(number=w3877, width (-)=i16 6, precision (6)=i16 2) -> (F-format string=w3876:string)  [unwired: 1 in]
                n3045 = Number To Fractional String(number=w3891, width (-)=i16 6, precision (6)=i16 2) -> (F-format string=w3897:string)  [unwired: 1 in]
                n3046 = Number To Fractional String(number=w3892, width (-)=i16 6, precision (6)=i16 2) -> (F-format string=w3890:string)  [unwired: 1 in]
                n3047 = Number To Fractional String(number=w3896, width (-)=i16 6, precision (6)=i16 2) -> (F-format string=w3895:string)  [unwired: 1 in]
                n3048 = Number To Fractional String(number=w3888, width (-)=i16 6, precision (6)=i16 2) -> (F-format string=w3886:string)  [unwired: 1 in]
                n3049 = Number To Fractional String(number=w3889, width (-)=i16 6, precision (6)=i16 2) -> (F-format string=w3887:string)  [unwired: 1 in]
                n3050 = Number To Fractional String(number=w3900, width (-)=i16 6, precision (6)=i16 2) -> (F-format string=w3901:string)  [unwired: 1 in]
                n3051 = Number To Fractional String(number=w3904, precision (6)=i16 2) -> (F-format string=w3905:string)  [unwired: 2 in]
                n3052 = local read "s.NO"() -> (w3824:string)
                n3053 = Concatenate Strings("=" ("string"), w3830) -> (w3829:string)
                n3054 = Concatenate Strings("S.No," ("string"), "                                       Parameters" ("string")) -> (w3835:string)
                n3055 = Concatenate Strings(w3902, w3861, w3876, w3902, w3858, w3897, w3902, w3857, w3890, w3902, w3853, w3895, w3902, w3851, w3886, w3902, w3848, w3887, w3902, w3845, w3901, w3902, w3842, w3905) -> (w3864:string)
                n3056 = Concatenate Strings(w3834, "," ("string"), w3822, w3824, w3823, w3906, w3909, w3823, w3907, w3908, w3834) -> (w3832:string)
                n3057 = local read "Tested by"() -> (w3838:string)
                n3058 = local read "String 33"() -> (w3839:string)
                n3059 = Concatenate Strings("," ("string"), "                                                                             " ("string")) -> (w3827:string)
                n3060 = Concatenate Strings(w3829, w3825, w3832, w3825, w3835, w3864, w3825, w3827, w3839, w3838) -> (→"export":string)
                n3061 = String To Path(string=w3866) -> (path=w3873:path)
                n3062 = local read "export"() -> (w3868:string)
                n3063 = call <vilib>:"Write Characters To File.vi"("append to file? (new file:F)"=FALSE, "character string"=w3868, "file path (dialog if empty)"=w3873) -> ()  [unwired: 2 in, 1 out]
              }
            }
          }
          frame Enabled {
          }
        }
        n3064 = case shown="True" "OK Button 17" {
          frame False {
          }
          frame True {
            (unwired) 0  # existing file
            w4126 = "Choose a datalog file to open"  # prompt
            n3065 = local write "OK Button 17"(FALSE ("OK Button 17")) -> ()
            n3066 = local read "String"() -> (w4121:string)
            n3067 = String To Path(string=w4121) -> (path=w4122:path)
            n3068 = File Dialog(6:"*.duf" ("pattern"), 7:w4126, 11:w4122) -> (0:w4113:errorcluster, 3:w4132:path)  [unwired: 4 in, 2 out]
            n3069 = Unbundle(w4113) -> ()  [unwired: 3 out]
            n3070 = Open/Create/Replace File "Open File"(file path (use dialog)=w4132) -> (refnum out=w4124:refnum<file>)  [unwired: 5 in, 2 out]
            n3071 = Strip Path(path=w4132) -> (name=w4130:string)  [unwired: 1 out]
            n3072 = Path To String(path=w4132) -> (string=w4115:string)
            n3073 = while {
              tunnel: w4124 -> [w4136]
              i -> [w4133]
              stop <- w4134 continue-if-true
              (unwired) TRUE ("line mode (F)")
              n3074 = Read from Text File "Read File"(file (use dialog)=w4136) -> (text=w4135:string)  [unwired: 3 in, 3 out]
              n3075 = local write "Numeric 16"(w4133) -> ()
              n3076 = String Length(string=w4135) -> (length=w4138:i32)
              n3077 = Greater?(x=w4138, y=1) -> (0:w4134:bool)
            }
            n3078 = local write "String 29"(w4115) -> ()
            n3079 = Search and Replace String(input string=w4115, search string=".duf", replace string=".dgf" ("replace string (\"\")")) -> (result string=→"String Indicator 4":string)  [unwired: 5 in, 3 out]
            n3080 = Match Pattern(string=w4130, regular expression=".dwm") -> (before substring=w4114:string)  [unwired: 1 in, 3 out]
            "String Indicator" <- w4114
            n3081 = Match Pattern(string=w4115, regular expression=".dwm" ("substring (\"\")")) -> (before substring=w4116:string)  [unwired: 1 in, 3 out]
            "String Indicator 3" <- w4116
            n3082 = local write "TITTLE 2"(w4114) -> ()
            n3083 = String To Path(string=w4116) -> (path=w4123:path)
            "path" <- w4123
            n3084 = call <vilib>:"Read Characters From File.vi"("file path (dialog if empty)"=w4123, "start of read offset (chars.:0)"=60 ("start of read offset (chars.: 0)")) -> ("character string"=→"String Indicator 2":string)  [unwired: 4 in, 3 out]
          }
        }
        n3085 = call <vilib>:"Query Available Printers.vi"() -> ("system configured printers"=w3815:string[])  [unwired: 9 in, 2 out]
        "System Configured Printers 2" <- w3815
        n3086 = local read "OK Button 16"() -> (w3812:bool)
        n3087 = case shown="True" "OK Button 16" {
          frame False {
          }
          frame True {
            n3088 = stacked-sequence {
              frame #0 {
                n3089 = local read "Numeric 16"() -> (w4140:i32)
                n3090 = local write "Numeric 10"(w4140) -> ()
              }
              frame #1 {
                n3091 = local read "String 29"() -> (w4143:string)
                n3092 = String To Path(string=w4143) -> (path=w4142:path)
                n3093 = Open/Create/Replace File "Open File"(file path (use dialog)=w4142) -> (refnum out=w4144:refnum<file>)  [unwired: 5 in, 2 out]
                n3094 = for {
                  N: 16 -> [_]
                  tunnel: w4144 -> [w4151]
                  i -> [w4147]
                  (unwired) TRUE ("line mode (F)")
                  n3095 = Read from Text File "Read File"(file (use dialog)=w4151) -> (text=w4145:string)  [unwired: 3 in, 3 out]
                  n3096 = Match Pattern(string=w4145, regular expression="(") -> (after substring=w4150:string)  [unwired: 1 in, 3 out]
                  n3097 = Match Pattern(string=w4150, regular expression=")") -> (before substring=w4146:string)  [unwired: 1 in, 3 out]
                  n3098 = case shown="1" w4147 {
                    tunnel: w4146 -> [w4152 w4153 _ _ w4154 w4155 w4156 w4158 w4160 w4162 w4164 w4166 w4168 w4170 _]
                    tunnel: w4145 -> [_ _ _ _ _ _ _ _ _ _ _ _ _ _ _]
                    frame 0 {
                      "TITTLE" <- w4152
                    }
                    frame 1 {
                      "Sample ID" <- w4153
                    }
                    frame 2 {
                    }
                    frame 3 {
                    }
                    frame 4 {
                      "Test Date" <- w4154
                    }
                    frame 5 {
                      "Tested by" <- w4155
                    }
                    frame 6 {
                      n3099 = Fract/Exp String To Number(string=w4156) -> (number=→"Humidity before test 2":dbl)  [unwired: 3 in, 1 out]
                    }
                    frame 7 {
                      n3100 = Fract/Exp String To Number(string=w4158) -> (number=→"Temperature before test 2":dbl)  [unwired: 3 in, 1 out]
                    }
                    frame 8 {
                      n3101 = Fract/Exp String To Number(string=w4160) -> (number=→"Humidity after test 2":dbl)  [unwired: 3 in, 1 out]
                    }
                    frame 9 {
                      n3102 = Fract/Exp String To Number(string=w4162) -> (number=→"Temperature after test 2":dbl)  [unwired: 3 in, 1 out]
                    }
                    frame 10 {
                      n3103 = Fract/Exp String To Number(string=w4164) -> (number=→"MWSD 2":dbl)  [unwired: 3 in, 1 out]
                    }
                    frame 11 {
                      n3104 = Fract/Exp String To Number(string=w4166) -> (number=→"AVP 2":dbl)  [unwired: 3 in, 1 out]
                    }
                    frame 12 {
                      n3105 = Fract/Exp String To Number(string=w4168) -> (number=→"HCF 2":dbl)  [unwired: 3 in, 1 out]
                    }
                    frame 13 {
                      n3106 = Fract/Exp String To Number(string=w4170) -> (number=→"WS1.4 2":dbl)  [unwired: 3 in, 1 out]
                    }
                    frame 14, Default {
                    }
                  }
                }
              }
              frame #2 {
              }
            }
            n3107 = local write "OK Button 16"(FALSE ("OK Button 13")) -> ()
          }
        }
        n3108 = Index Array(array=w3815, index="Select Printer 3") -> (element=w3817:string)
        "Selected Printer" <- w3817
        n3109 = case shown="True" w3812 {
          frame False {
          }
          frame True {
            n3110 = flat-sequence {
              frame #0 {
              }
              frame #1 {
                n3111 = Wait (ms)(milliseconds to wait=u32 100) -> ()  [unwired: 1 out]
              }
              frame #2 {
                n3112 = local write "OK Button 16"(FALSE ("Print 3")) -> ()
              }
            }
          }
        }
        n3113 = case shown="True" "Print" {
          tunnel: w3817 -> [_ w4109]
          frame False {
          }
          frame True {
            (unwired) i16 6 ("width (-)")
            (unwired) "TESTED BY : "
            (unwired) "TESTED DATE :"
            (unwired) "SAMPLE ID : "
            (unwired) "SAMPLE DESIGN : "
            w4067 = "\r"
            w4084 = "\r"
            # "add image"
            n3114 = local read "Sample ID"() -> (w4057:string)
            n3115 = local read "Tested by"() -> (w4060:string)
            n3116 = local read "String 34"() -> (w4047:string)
            n3117 = local read "String 45"() -> (w4027:string)
            n3118 = local read "String 35"() -> (w4042:string)
            n3119 = local read "String 37"() -> (w4040:string)
            n3120 = local read "String 32"() -> (w4062:string)
            n3121 = local read "String 36"() -> (w4037:string)
            n3122 = local read "String 31"() -> (w4061:string)
            n3123 = local read "Test Date"() -> (w4058:string)
            n3124 = local read "String 33"() -> (w4063:string)
            n3125 = local read "String 38"() -> (w4033:string)
            n3126 = local read "String 39"() -> (w4030:string)
            n3127 = local write "Print"(FALSE ("Print FF")) -> ()
            n3128 = local read "S 39"() -> (w4045:string)
            n3129 = local read "S 38"() -> (w4052:string)
            n3130 = local read "Temperature before test 2"() -> (w4083:dbl)
            n3131 = local read "Temperature after test 2"() -> (w4073:dbl)
            n3132 = local read "Humidity before test 2"() -> (w4098:dbl)
            n3133 = local read "Humidity after test 2"() -> (w4082:dbl)
            n3134 = local read "MWSD 2"() -> (w4087:dbl)
            n3135 = local read "WS1.4 2"() -> (w4065:dbl)
            n3136 = Concatenate Strings("2)" ("string"), w4047) -> (w4048:string)
            n3137 = Concatenate Strings("3)" ("string"), w4045) -> (w4046:string)
            n3138 = Concatenate Strings("1)" ("string"), w4052) -> (w4051:string)
            n3139 = Concatenate Strings("4)" ("string"), w4042) -> (w4043:string)
            n3140 = Concatenate Strings("5)" ("string"), w4040) -> (w4039:string)
            n3141 = Concatenate Strings("6)" ("string"), w4037) -> (w4036:string)
            n3142 = Concatenate Strings("7)" ("string"), w4033) -> (w4034:string)
            n3143 = Concatenate Strings("8)" ("string"), w4030) -> (w4031:string)
            n3144 = local read "HCF 2"() -> (w4069:dbl)
            n3145 = local read "AVP 2"() -> (w4086:dbl)
            n3146 = local read "s.NO"() -> (w4028:string)
            n3147 = call <vilib>:"New Report.vi"("report type"=enum16{"Standard Report", "HTML"}."Standard Report") -> ("report out"=w4107:refnum<class "NI_report.lvclass">, "error out"=w4106:errorcluster)  [unwired: 13 in]
            n3148 = local read "TITTLE"() -> (w4059:string)
            n3149 = Concatenate Strings(w4084, w4027, w4028, w4084, w4062, w4057, w4084, w4061, w4058, w4084, w4063, w4060, w4084) -> (w4077:string)
            "test by" <- w4077
            n3150 = Number To Fractional String(number=w4083, width (-)=i16 6, precision (6)=i16 2) -> (F-format string=w4072:string)  [unwired: 1 in]
            n3151 = Number To Fractional String(number=w4082, width (-)=i16 6, precision (6)=i16 2) -> (F-format string=w4085:string)  [unwired: 1 in]
            n3152 = Number To Fractional String(number=w4098, width (-)=i16 6, precision (6)=i16 2) -> (F-format string=w4103:string)  [unwired: 1 in]
            n3153 = Number To Fractional String(number=w4087, width (-)=i16 6, precision (6)=i16 2) -> (F-format string=w4089:string)  [unwired: 1 in]
            n3154 = Number To Fractional String(number=w4073, width (-)=i16 6, precision (6)=i16 2) -> (F-format string=w4074:string)  [unwired: 1 in]
            n3155 = Number To Fractional String(number=w4086, width (-)=i16 6, precision (6)=i16 2) -> (F-format string=w4088:string)  [unwired: 1 in]
            n3156 = Number To Fractional String(number=w4069, width (-)=i16 6, precision (6)=i16 2) -> (F-format string=w4068:string)  [unwired: 1 in]
            n3157 = Number To Fractional String(number=w4065, precision (6)=i16 2) -> (F-format string=w4064:string)  [unwired: 2 in]
            n3158 = call-dynamic "Set Report Header Text.vi"("report in"=w4107, "center header text"=w4059, "error in (no error)"=w4106) -> ("report out"=w4078:refnum<class "NI_report.lvclass">, "error out"=w4079:errorcluster)  [unwired: 11 in]
            n3159 = Concatenate Strings(w4067, w4051, w4103, w4067, w4048, w4072, w4067, w4046, w4085, w4067, w4043, w4074, w4067, w4039, w4089, w4067, w4036, w4088, w4067, w4034, w4068, w4067, w4031, w4064) -> (w4055:string)
            "export 2" <- w4055
            n3160 = call-poly <vilib>:"Append Report Text.vi"("report in"=w4078, "text"=w4077, "error in (no error)"=w4079) -> ("report out"=w4081:refnum<class "NI_report.lvclass">, "error out"=w4080:errorcluster)  [unwired: 9 in, 2 out]
            n3161 = local read "test by"() -> (w4054:string)
            n3162 = local read "TITTLE"() -> (w4056:string)
            n3163 = call-poly <vilib>:"Append Report Text.vi"("report in"=w4081, "error in (no error)"=w4080) -> ("report out"=w4102:refnum<class "NI_report.lvclass">, "error out"=w4100:errorcluster)  [unwired: 10 in, 2 out]
            n3164 = Concatenate Strings(w4056, w4055, w4054) -> (→"output":string)
            n3165 = call-poly <vilib>:"Append Report Text.vi"("report in"=w4102, "text"=w4055, "error in (no error)"=w4100) -> ("report out"=w4101:refnum<class "NI_report.lvclass">, "error out"=w4099:errorcluster)  [unwired: 9 in, 2 out]
            n3166 = call-dynamic "Print Report.vi"("report in"=w4101, "printer name (default)"=w4109, "error in (no error)"=w4099) -> ("report out"=w4111:refnum<class "NI_report.lvclass">, "error out"=w4112:errorcluster)  [unwired: 11 in]
            n3167 = call-dynamic "Dispose Report.vi"("report in"=w4111, "error in (no error)"=w4112) -> ()  [unwired: 13 in, 1 out]
          }
        }
        n3168 = case shown="True" "Print 2" {
          frame False {
          }
          frame True {
            n3169 = flat-sequence {
              frame #0 {
                n3170 = local read "s.NO"() -> (→"s.NO 2":string)
                n3171 = Wait (ms)(milliseconds to wait=u32 20) -> ()  [unwired: 1 out]
                n3172 = local read "Sample ID  3"() -> (→"Sample ID  6":string)
                n3173 = local read "Sample ID  4"() -> (→"Sample ID  7":string)
                n3174 = local read "Sample ID"() -> (→"Sample ID  2":string)
                n3175 = local read "Tested by"() -> (→"Tested by 2":string)
                n3176 = local read "Test Date"() -> (→"Test Date 2":string)
                n3177 = local read "Humidity after test 3"() -> (→"Humidity after test 4":dbl)
                n3178 = local read "Ref A Test Date :"() -> (→"TITTLE 4":string)
                n3179 = local read "Temperature before test 3"() -> (w3934:dbl)
                n3180 = local read "Temperature before test 3"() -> (→"Temperature after test 5":dbl)
                n3181 = local read "Temperature after test 3"() -> (→"Temperature after test 4":dbl)
                n3182 = local read "Humidity before test 3"() -> (→"Humidity before test 4":dbl)
                n3183 = local write "Temperature before test 3"(w3934) -> ()
                n3184 = local read "image data"() -> (w3925:T2)
                n3185 = String To Path(string="C:\\LAB-IQ\\im\\Temp_resized.jpg") -> (path=w3926:path)
                "path 2" <- w3926
                n3186 = call <vilib>:"Write JPEG File.vi"("image data"=w3925, "path to JPEG file"=w3926) -> ()  [unwired: 8 in, 2 out]
                "Ref A Test Date :" <- "Ref A Test Date :"
                "Ref B Test Date :" <- "Ref B Test Date :"
                "Ref B Scar Value :" <- "Ref B Scar Value :"
                "Ref A Scar Value :" <- "Ref A Scar Value :"
              }
              frame #1 {
                (unwired) HTML_Report_Image_Alignment."MIDDLE" ("alignment (default)")
                w3962 = u16 0 items=["portrait", "landscape"] ("orientation (portrait)")
                (unwired) HTML_Report_Image_Alignment."ABSMIDDLE" ("alignment (default)")
                (unwired) "TESTED BY : "
                (unwired) "TESTED DATE :"
                (unwired) "SAMPLE ID : "
                (unwired) "SAMPLE DESIGN : "
                w3995 = "\r"
                # "add image"
                n3187 = Wait (ms)(milliseconds to wait=u32 20) -> ()  [unwired: 1 out]
                n3188 = local read "Sample ID  2"() -> (w3988:string)
                n3189 = local read "Wear Scar X"() -> (w3960:dbl)
                "Length ( microns ) 2" <- w3960
                n3190 = local read "Wear Scar Y"() -> (w3959:dbl)
                "Wear Scar Y ( microns ) :" <- w3959
                n3191 = local read "Test Date 2"() -> (w3989:string)
                n3192 = local read "Tested by 2"() -> (w3990:string)
                n3193 = local read "String 46"() -> (w3986:string)
                n3194 = local read "String 48"() -> (w3992:string)
                n3195 = local read "String 47"() -> (w3991:string)
                n3196 = local read "String 49"() -> (w3993:string)
                n3197 = local read "String 10"() -> (w3946:string)
                n3198 = local read "s.NO 2"() -> (w3987:string)
                n3199 = Add(x=w3960, y=w3959) -> (x+y=w3958:dbl)
                n3200 = call <vilib>:"New Report.vi"("report type"=enum16{"Standard Report", "HTML"}."HTML") -> ("report out"=w3966:refnum<class "NI_report.lvclass">, "error out"=w3964:errorcluster)  [unwired: 13 in]
                n3201 = Concatenate Strings(w3995, w3986, w3987, w3995, w3992, w3988, w3995, w3991, w3989, w3995, w3993, w3990, w3995) -> (→"test by 2":string)
                n3202 = Concatenate Strings("C:\\LAB-IQ\\Data\\" ("string"), w3946, ".jpg" ("string")) -> ()  [unwired: 1 out]
                n3203 = Divide(x=w3958, y=2.0) -> (x/y=→"Mean Wear ( microns) :":dbl)
                n3204 = call-dynamic "Set Report Orientation.vi"("report in"=w3966, "orientation (portrait)"=w3962, "error in (no error)"=w3964) -> ("report out"=w3965:refnum<class "NI_report.lvclass">, "error out"=w3963:errorcluster)  [unwired: 11 in]
                n3205 = for {
                  N: 5 -> [_]
                  tunnel: w3965 -> [w4016]
                  tunnel: [w4015] -> w3944
                  tunnel: w3963 -> [w4014]
                  tunnel: [w4013] -> w3943